vi "HFRR ADV v041.vi"() -> ()   [LabVIEW 2025] (continued)
                n3153 = for {
                  N: 1 -> [_]
                  tunnel: [w3970] -> w3918
                  tunnel: [w3969] -> w3917
                  tunnel: w3932 -> [w3968]
                  tunnel: w3931 -> [w3967]
                  n3154 = call-dynamic "New Report Line.vi"("report in"=w3968, "error in (no error)"=w3967) -> ("report out"=w3970:refnum<class "NI_report.lvclass">, "error out"=w3969:errorcluster)  [unwired: 12 in]
                }
                n3155 = for {
                  N: 2 -> [_]
                  tunnel: [w3962] -> w3924
                  tunnel: [w3961] -> w3923
                  tunnel: w3918 -> [w3960]
                  tunnel: w3917 -> [w3959]
                  n3156 = call-dynamic "New Report Line.vi"("report in"=w3960, "error in (no error)"=w3959) -> ("report out"=w3962:refnum<class "NI_report.lvclass">, "error out"=w3961:errorcluster)  [unwired: 12 in]
                }
                n3157 = for {
                  N: 25 -> [_]
                  tunnel: w3924 -> [w3958]
                  tunnel: w3923 -> [w3956]
                  tunnel: [w3957] -> w3927
                  tunnel: [w3955] -> w3926
                  n3158 = call-dynamic "Set Report Tab Width.vi"("report in"=w3958, "error in (no error)"=w3956) -> ("report out"=w3957:refnum<class "NI_report.lvclass">, "error out"=w3955:errorcluster)  [unwired: 12 in]
                }
                n3159 = control-ref of="Tab Control 9"() -> (w3922:refnum<vi>)
                n3160 = call-dynamic "Append Control Image to Report.vi"("report in"=w3927, "alignment (default)"=HTML_Report_Image_Alignment."ABSMIDDLE", "ctrl reference"=w3922, "error in (no error)"=w3926) -> ("report out"=w3921:refnum<class "NI_report.lvclass">, "error out"=w3920:errorcluster)  [unwired: 8 in, 2 out]
                n3161 = for {
                  N: 3 -> [_]
                  tunnel: [w3954] -> w3905
                  tunnel: [w3953] -> w3904
                  tunnel: w3921 -> [w3952]
                  tunnel: w3920 -> [w3951]
                  n3162 = call-dynamic "New Report Line.vi"("report in"=w3952, "error in (no error)"=w3951) -> ("report out"=w3954:refnum<class "NI_report.lvclass">, "error out"=w3953:errorcluster)  [unwired: 12 in]
                }
                n3163 = for {
                  N: 100 -> [_]
                  tunnel: w3905 -> [w3950]
                  tunnel: w3904 -> [w3948]
                  tunnel: [w3949] -> w3901
                  tunnel: [w3947] -> w3899
                  n3164 = call-dynamic "Set Report Tab Width.vi"("report in"=w3950, "error in (no error)"=w3948) -> ("report out"=w3949:refnum<class "NI_report.lvclass">, "error out"=w3947:errorcluster)  [unwired: 12 in]
                }
                n3165 = String To Path(string="C:\\LAB-IQ\\im\\Temp_resized.jpg") -> (path=w3891:path)
                n3166 = call-poly <vilib>:"Append Image to Report.vi"("report in"=w3901, "path or URL of image"=w3891, "error in (no error)"=w3899) -> ("report out"=w3900:refnum<class "NI_report.lvclass">, "error out"=w3898:errorcluster)  [unwired: 9 in, 2 out]
                n3167 = call-poly <vilib>:"Open HTML Report in Browser.vi"("report in"=w3900, "error in (no error)"=w3898) -> ("report out"=w3935:refnum<class "NI_report.lvclass">, "error out"=w3934:errorcluster)  [unwired: 11 in, 1 out]
                n3168 = call-dynamic "Dispose Report.vi"("report in"=w3935, "error in (no error)"=w3934) -> ()  [unwired: 13 in, 1 out]
              }
              frame #2 {
              }
              frame #3 {
                n3169 = disable-structure shown="Disabled" {
                  frame Disabled {
                    n3170 = local read "String 10"() -> (w3975:string)
                    n3171 = Concatenate Strings("C:\\LAB-IQ-NXT\\Data\\" ("string"), w3975, ".jpg" ("string")) -> (w3973:string)
                    n3172 = String To Path(string=w3973) -> (path=w3972:path)
                    n3173 = Delete(path (use dialog)=w3972) -> ()  [unwired: 4 in, 3 out]
                  }
                  frame Enabled {
                  }
                }
                n3174 = local write "Print 2"(FALSE ("Print")) -> ()
              }
            }
          }
        }
      }
    }
    n3175 = Wait (ms)(milliseconds to wait=u32 50) -> ()  [unwired: 1 out]
    n3176 = Wait (ms)(milliseconds to wait=u32 50) -> ()  [unwired: 1 out]
    n3177 = local read "Quit"() -> (w2317:bool)
  }
  n3178 = VISA Close(VISA resource name=w43, error in (no error)=w42) -> ()  [unwired: 1 out]
  n3179 = while {
    stop <- w4126 stop-if-true
    n3180 = local read "Auto Start Test"() -> (w4124:bool)
    n3181 = local read "RUN"() -> (w4123:bool)
    n3182 = Wait (ms)(milliseconds to wait=u32 1000) -> ()  [unwired: 1 out]
    n3183 = Or(x=w4123, y=w4124) -> (x .or. y?=w4122:bool)
    n3184 = case shown="True" w4122 {
      frame False {
      }
      frame True {
        n3185 = local read "LVDT STROKE Actual"() -> (w4127:dbl)
        n3186 = In Range and Coerce(upper limit=1.2, x=w4127, lower limit=0.6) -> (In Range?=w4130:bool)  [unwired: 1 out]
        n3187 = call-poly <vilib>:"Random Number (Range).vi"("lower bound (0)"=0.998 ("upper bound (100)"), "upper bound (100)"=1.003) -> ("number"=w4128:dbl)  [unwired: 9 in]
        n3188 = case shown="True" w4130 {
          tunnel: [w4135 w4136] -> w4129
          tunnel: w4128 -> [_ w4136]
          tunnel: w4127 -> [w4135 _]
          frame False {
          }
          frame True {
          }
        }
        "LVDT STROKE DISPLAY" <- w4129
      }
    }
    n3189 = local read "Quit"() -> (w4126:bool)
  }
  n3190 = while {
    tunnel: [w4153] -> w51
    shift-right: [w4146] -> _
    shift-left: 0.0 -> [w4149]
    shift-right: [w4145] -> _
    shift-left: 0.0 -> [w4148]
    shift-right: [w4144] -> _
    shift-left: 100.0 ("vc_cmd") -> [w4147]
    stop <- w4153 stop-if-true
    # "PID LOGIC"
    n3191 = local read "run test Calibration"() -> (w4141:bool)
    n3192 = local read "RUN"() -> (w4151:bool)
    n3193 = local read "Auto Start Temp"() -> (w4142:bool)
    n3194 = local read "Auto Start Test"() -> (w4150:bool)
    n3195 = local read "START TEMP"() -> (w4140:bool)
    n3196 = And(x=w4142, y=w4150) -> (x .and. y?=w4143:bool)
    n3197 = Or(x=w4151, y=w4143) -> (x .or. y?=w4152:bool)
    n3198 = And(x=w4152, y=w4140) -> (x .and. y?=w4139:bool)
    n3199 = And(x=w4141, y=w4140) -> (x .and. y?=w4138:bool)
    n3200 = Or(x=w4138, y=w4139) -> (x .or. y?=w4137:bool)
    n3201 = Wait (ms)(milliseconds to wait="milliseconds to wait") -> ()  [unwired: 1 out]
    n3202 = case shown="True" w4137 {
      tunnel: [400.0 ("out_vc_cmd") w4172] -> w4144
      tunnel: [w4156 w4174] -> w4145
      tunnel: [w4156 w4173] -> w4146
      tunnel: w4149 -> [_ w4163]
      tunnel: w4148 -> [_ w4162]
      tunnel: w4147 -> [_ w4161]
      tunnel: w4141 -> [_ w4157]
      frame False {
        w4156 = 0.0 ("error_out")
      }
      frame True {
        n3203 = case shown="True" w4157 {
          tunnel: [w4181 1.0] -> w4159
          frame False {
            n3204 = local read "Set Strk"() -> (w4180:dbl)
            n3205 = Add(x=w4180, y="Add up Stroke") -> (x+y=w4181:dbl)
          }
          frame True {
          }
        }
        n3206 = local read "LVDT STROKE"() -> (w4158:dbl)
        n3207 = formula code="// Zero-Hardcode Explicit Positional-Form PID Engine\n// Inputs: target_stroke, measured_stroke, dt, prev_error, integral_accumulator_in, prev_vc_cmd\n//         kp, ki, kd, max_step_change, max_amplitude, min_amplitude, startup_cmd\n// Outputs: vc_cmd, error_out, out_error, integral_accumulator_out, out_vc_cmd\n\n// 1. Calculate Tracking Error\nfloat current_error = target_stroke - measured_stroke;\nerror_out = current_error;\n\n// 2. Compute Proportional Term\nfloat p_term = kp * current_error;\n\n// 3. Compute Derivative Term\nfloat d_term = 0.0;\nif (dt > 0.0) {\n    d_term = kd * ((current_error - prev_error) / dt);\n}\n\n// 4. Update and Accumulate Integral Term\nfloat current_integral = integral_accumulator_in + (current_error * dt);\nfloat i_term = ki * current_integral;\n\n// 5. Calculate Ideal Target Command (Anchored by startup baseline)\nfloat ideal_command = startup_cmd + p_term + i_term + d_term;\n\n// 6. Apply Loop Rate Limiting FIRST \n// (Forces the command to climb gradually from prev_vc_cmd instead of jumping straight to max)\nfloat raw_adjustment = ideal_command - prev_vc_cmd;\n\nif (raw_adjustment > max_step_change) {\n    raw_adjustment = max_step_change;\n} else if (raw_adjustment < -max_step_change) {\n    raw_adjustment = -max_step_change;\n}\n\nfloat next_vc_cmd = prev_vc_cmd + raw_adjustment;\n\n// 7. Anti-Windup Protection & Final Output Safety Safeguard Clamping\n// (Back-calculating based on what we are ACTUALLY outputting)\nif (next_vc_cmd > max_amplitude) {\n    float excess = next_vc_cmd - max_amplitude;\n    if (ki > 0.0) {\n        current_integral -= excess / ki;\n    }\n    next_vc_cmd = max_amplitude;\n} else if (next_vc_cmd < min_amplitude) {\n    float excess = next_vc_cmd - min_amplitude;\n    if (ki > 0.0) {\n        current_integral -= excess / ki;\n    }\n    next_vc_cmd = min_amplitude;\n}\n\n// 8. Map to Shift Registers for memory persistence\nvc_cmd = next_vc_cmd;\nout_error = current_error;                   \nintegral_accumulator_out = current_integral;  \nout_vc_cmd = next_vc_cmd;"("target_stroke"=w4159, "measured_stroke"=w4158, "dt"="dt", "integral_accumulator_in"=w4162, "prev_error"=w4163, "prev_vc_cmd"=w4161, "kp"="kp", "ki"="ki", "kd"="kd", "max_step_change"="max_step_change", "max_amplitude"="max_amplitude", "min_amplitude"="min_amplitude", "startup_cmd"="startup_cmd") -> ("vc_cmd"=w4178:dbl, "out_error"=w4173:dbl, "integral_accumulator_out"=w4174:dbl, "out_vc_cmd"=w4172:dbl)  [unwired: 1 out]
        "output Vpp" <- w4178
        n3208 = Number To Fractional String(number=w4178, precision (6)=i16 1) -> (F-format string=w4176:string)  [unwired: 2 in]
        n3209 = Concatenate Strings("DAC;" ("string"), w4176) -> (w4160:string)
        n3210 = local write "Due Write"(w4160) -> ()
        "prev_error" <- w4163
        "integral_accumulator_in" <- w4162
        "prev_vc_cmd" <- w4161
      }
    }
    n3211 = local read "Quit"() -> (w4153:bool)
  }
  n3212 = Or(x=w47, y=w46) -> (x .or. y?=w48:bool)
  n3213 = Or(x=w44, y=w48) -> (x .or. y?=w53:bool)
  n3214 = control-ref of="new picture"() -> ()  [unwired: 1 out]
  n3215 = Or(x=w56, y=w53) -> (x .or. y?=w50:bool)
  n3216 = Or(x=w50, y=w51) -> (x .or. y?=w45:bool)
  n3217 = while {
    tunnel: [w4183] -> w55
    i -> [w4190]
    stop <- w4183 stop-if-true
    n3218 = local read "Quit"() -> (w4183:bool)
    n3219 = Equal To 0?(x=w4190) -> (x = 0?=w4188:bool)
    n3220 = call "Elapsed Time3"("Time Target (s)"=45.0, "Auto Reset"=TRUE) -> ("Time has Elapsed"=w4187:bool)  [unwired: 10 in, 7 out]
    n3221 = Wait (ms)(milliseconds to wait=u32 50) -> ()  [unwired: 1 out]
    n3222 = Or(x=w4187, y=w4188) -> (x .or. y?=w4189:bool)
    n3223 = case shown="True" w4189 {
      frame False {
      }
      frame True {
        n3224 = call <vilib>:"System Exec.vi"("run minimized? (F)"=TRUE, "error in (no error)"="error in (no error)", "command line"="powercfg.exe -change -monitor-timeout-ac 0") -> ("error out"=w4201:errorcluster)  [unwired: 5 in, 3 out]
        n3225 = call <vilib>:"System Exec.vi"("run minimized? (F)"=TRUE, "error in (no error)"=w4201, "command line"="powercfg.exe -change -disk-timeout-ac 0") -> ("error out"=w4200:errorcluster)  [unwired: 5 in, 3 out]
        n3226 = call <vilib>:"System Exec.vi"("run minimized? (F)"=TRUE, "error in (no error)"=w4200, "command line"="powercfg.exe -change -standby-timeout-ac 0") -> ("error out"=w4199:errorcluster)  [unwired: 5 in, 3 out]
        n3227 = call <vilib>:"System Exec.vi"("run minimized? (F)"=TRUE, "error in (no error)"=w4199, "command line"="powercfg.exe -change -hibernate-timeout-ac 0") -> ("error out"=w4198:errorcluster)  [unwired: 5 in, 3 out]
        n3228 = call <vilib>:"Simple Error Handler.vi"("error in (no error)"=w4198) -> ("error out"=w4204:errorcluster)  [unwired: 4 in, 4 out]
        n3229 = call <vilib>:"Clear Errors.vi"("error in (no error)"=w4204) -> ("error out"=→"error out":errorcluster)  [unwired: 5 in, 1 out]
      }
    }
  }
  n3230 = Compound Arithmetic op=OR(w58, w45, w55) -> (w57:bool)
  n3231 = flat-sequence {
    tunnel: w57 -> [_]
    tunnel: [w4206] -> w27
    tunnel: w27 -> [_]
    frame #0 {
      n3232 = call "CLOSE CONNECTION.vi"() -> ("error out"=w4206:errorcluster)  [unwired: 11 in]
    }
    frame #1 {
      n3233 = Quit LabVIEW(quit? (T)=TRUE) -> ()
      n3234 = local write "Quit"(FALSE ("EXIT")) -> ()
    }
  }
  n3235 = property on="Heater Button" class="Bool (strict)"("Visible"=TRUE) -> ()  [unwired: 2 in, 2 out]
  n3236 = while {
    tunnel: [w4213] -> _
    i -> [w4213]
    stop <- w4209 stop-if-true
    # "Langauage selection"
    n3237 = Equal?(x="Lan flag", y=22.0) -> ()  [unwired: 1 out]
    n3238 = disable-structure shown="Disabled" {
      frame Disabled {
        n3239 = stacked-sequence {
          frame #0 {
            n3240 = case shown="\"Russian\"" "Language Selection" {
              tunnel: [0 1] -> w4215
              frame "English", Default {
              }
              frame "Russian" {
              }
            }
            n3241 = for {
              N: 130 -> [_]
              tunnel: "Table" -> [w4224]
              tunnel: w4215 -> [w4223]
              i -> [w4222]
              n3242 = Index Array(array=w4224, index (row)=w4222, index (col)=w4223) -> (element=w4221:string)
              n3243 = case shown="1" w4222 {
                tunnel: w4221 -> [w4225 w4226 _ w4227 w4228 w4229 w4230 w4231 w4232 w4233 w4234 w4235 w4236 w4237 w4238 w4239 w4240 w4241 w4242 w4243 w4244 w4245 w4246 w4247 w4248 w4249 w4250 w4251 w4252 _ _ w4253 w4254 w4255 w4256 w4257 w4258 w4267 w4274 w4281 w4288 w4292 w4295 w4298 w4300 w4302 w4303 w4304 w4305 w4306 w4307 w4308 w4309 w4310 w4311 w4312 w4313 w4314 w4315 w4316 w4317 w4318 w4319 w4320 w4321 w4322 w4323 w4324 w4325 w4326 w4327 w4328 w4329 w4330 w4331 w4332 w4333 w4334 w4335 w4336 w4337 w4338 w4339 w4340 w4341 w4342 w4343 w4344 w4345 w4346 w4347 w4348 w4349 w4350 w4351 w4352 w4353 w4354 w4355 w4356 w4357 w4358 w4359 w4360 w4361 _ w4362 w4363 w4364 w4365 w4366 w4367 w4368 w4369 w4370 w4371 w4372 w4373 w4374 _ w4375 w4376 w4377 w4378 w4379 w4380 _]
                frame 0 {
                  n3244 = local write "S"(w4225) -> ()
                }
                frame 1 {
                  n3245 = local write "S 2"(w4226) -> ()
                }
                frame 2 {
                }
                frame 3 {
                  n3246 = local write "S 4"(w4227) -> ()
                }
                frame 4 {
                  n3247 = property on="FILE" class="Str"("Caption.Text"=w4228) -> ()  [unwired: 2 in, 2 out]
                }
                frame 5 {
                  n3248 = property on="Fuel Discription :" class="Str"("Caption.Text"=w4229) -> ()  [unwired: 2 in, 2 out]
                }
                frame 6 {
                  n3249 = property on="Remarks :" class="Str"("Caption.Text"=w4230) -> ()  [unwired: 2 in, 2 out]
                }
                frame 7 {
                  n3250 = property on="Save & Continue" class="Bool (strict)"("Boolean Text.Text"=w4231) -> ()  [unwired: 2 in, 2 out]
                }
                frame 8 {
                }
                frame 9 {
                  n3251 = property on="Set Hz" class="DigNum (strict)"("Caption.Text"=w4233) -> ()  [unwired: 2 in, 2 out]
                }
                frame 10 {
                }
                frame 11 {
                  n3252 = property on="NORMAL LOAD" class="DigNum (strict)"("Caption.Text"=w4235) -> ()  [unwired: 2 in, 2 out]
                }
                frame 12 {
                }
                frame 13 {
                  n3253 = property on="Set Temp" class="DigNum (strict)"("Caption.Text"=w4237) -> ()  [unwired: 2 in, 2 out]
                }
                frame 14 {
                  n3254 = local write "S 15"(w4238) -> ()
                }
                frame 15 {
                  n3255 = property on="Set Rh" class="DigNum (strict)"("Caption.Text"=w4239) -> ()  [unwired: 2 in, 2 out]
                }
                frame 16 {
                }
                frame 17 {
                  n3256 = local write "S 18"(w4241) -> ()
                }
                frame 18 {
                  "String 17" <- w4242
                }
                frame 19 {
                  n3257 = property on="test time" class="DigNum (strict)"("Caption.Text"=w4243) -> ()  [unwired: 2 in, 2 out]
                }
                frame 20 {
                  "String 18" <- w4244
                  "String 22" <- w4244
                }
                frame 21 {
                  n3258 = property on="Elapsed time" class="DigNum (strict)"("Caption.Text"=w4245) -> ()  [unwired: 2 in, 2 out]
                }
                frame 22 {
                  n3259 = property on="Samplingtime 2" class="DigNum (strict)"("Caption.Text"=w4246) -> ()  [unwired: 2 in, 2 out]
                }
                frame 23 {
                  "String 21" <- w4247
                }
                frame 24 {
                  n3260 = property on="Countdown" class="DigNum (strict)"("Caption.Text"=w4248) -> ()  [unwired: 2 in, 2 out]
                }
                frame 25 {
                  n3261 = property on="Countdown 2" class="DigNum (strict)"("Caption.Text"=w4249) -> ()  [unwired: 2 in, 2 out]
                }
                frame 26 {
                  n3262 = property on="Engage" class="Bool (strict)"("Boolean Text.Text"=w4250) -> ()  [unwired: 2 in, 2 out]
                }
                frame 27 {
                  n3263 = property on="Boolean  4" class="Bool (strict)"("Boolean Text.Text"=w4251) -> ()  [unwired: 2 in, 2 out]
                }
                frame 28 {
                  n3264 = property on="Test \nStatus" class="Bool (strict)"("Boolean Text.Text"=w4252) -> ()  [unwired: 2 in, 2 out]
                }
                frame 29 {
                }
                frame 30 {
                }
                frame 31 {
                }
                frame 32 {
                  n3265 = property on="RSTCOF" class="Bool"("Boolean Text.Text"=w4254) -> ()  [unwired: 2 in, 2 out]
                  n3266 = property on="RST FF" class="Bool"("Boolean Text.Text"=w4254) -> ()  [unwired: 2 in, 2 out]
                  n3267 = property on="RST TEMP" class="Bool"("Boolean Text.Text"=w4254) -> ()  [unwired: 2 in, 2 out]
                  n3268 = property on="RSTV1 3" class="Bool"("Boolean Text.Text"=w4254) -> ()  [unwired: 2 in, 2 out]
                  n3269 = property on="rstv2" class="Bool"("Boolean Text.Text"=w4254) -> ()  [unwired: 2 in, 2 out]
                  n3270 = property on="RSTV1 2" class="Bool"("Boolean Text.Text"=w4254) -> ()  [unwired: 2 in, 2 out]
                  n3271 = property on="RST CP" class="Bool"("Boolean Text.Text"=w4254) -> ()  [unwired: 2 in, 2 out]
                }
                frame 33 {
                  "S 61" <- w4255
                }
                frame 34 {
                  "String 23" <- w4256
                }
                frame 35 {
                  n3272 = property on="Rh Before" class="DigNum (strict)"("Caption.Text"=w4257) -> ()  [unwired: 2 in, 2 out]
                }
                frame 36 {
                  n3273 = Match Pattern(string=w4258, regular expression=",") -> (before substring=→"bs":string, after substring=→"as":string)  [unwired: 1 in, 2 out]
                  n3274 = property on="Rh After" class="DigNum (strict)"("Caption.Text"=w4258) -> ()  [unwired: 2 in, 2 out]
                }
                frame 37 {
                  n3275 = Match Pattern(string=w4267, regular expression=",") -> (before substring=w4266:string, after substring=w4265:string)  [unwired: 1 in, 2 out]
                  "bs" <- w4266
                  "as" <- w4265
                  n3276 = Concatenate Strings(w4266, w4265) -> (w4262:string)
                  n3277 = property on="Humidity before test 2" class="DigNum (strict)"("Caption.Text"=w4262) -> ()  [unwired: 2 in, 2 out]
                  n3278 = Concatenate Strings(w4262, "=" ("string")) -> (w4263:string)
                  n3279 = local write "S 38"(w4263) -> ()
                }
                frame 38 {
                  n3280 = Match Pattern(string=w4274, regular expression=",") -> (before substring=w4273:string, after substring=w4272:string)  [unwired: 1 in, 2 out]
                  "bs" <- w4273
                  "as" <- w4272
                  n3281 = Concatenate Strings(w4273, w4272) -> (w4269:string)
                  n3282 = property on="Humidity after test 2" class="DigNum (strict)"("Caption.Text"=w4269) -> ()  [unwired: 2 in, 2 out]
                  n3283 = Concatenate Strings(w4269, "=" ("string")) -> (w4271:string)
                  n3284 = local write "S 39"(w4271) -> ()
                }
                frame 39 {
                  n3285 = Match Pattern(string=w4281, regular expression=",") -> (before substring=w4280:string, after substring=w4279:string)  [unwired: 1 in, 2 out]
                  "bs" <- w4280
                  "as" <- w4279
                  n3286 = Concatenate Strings(w4280, w4279) -> (w4276:string)
                  n3287 = property on="Temperature before test 2" class="DigNum (strict)"("Caption.Text"=w4276) -> ()  [unwired: 2 in, 2 out]
                  n3288 = Concatenate Strings(w4276, "=" ("string")) -> (→"String 34":string)
                }
                frame 40 {
                  n3289 = Match Pattern(string=w4288, regular expression=",") -> (before substring=w4287:string, after substring=w4286:string)  [unwired: 1 in, 2 out]
                  "bs" <- w4287
                  "as" <- w4286
                  n3290 = Concatenate Strings(w4287, w4286) -> (w4283:string)
                  n3291 = property on="Temperature after test 2" class="DigNum (strict)"("Caption.Text"=w4283) -> ()  [unwired: 2 in, 2 out]
                  n3292 = Concatenate Strings(w4283, "=" ("string")) -> (→"String 35":string)
                  n3293 = property on="Temperature after test" class="DigNum (strict)"("Caption.Text"=w4283) -> ()  [unwired: 2 in, 2 out]
                }
                frame 41 {
                  n3294 = property on="AVP 2" class="DigNum (strict)"("Caption.Text"=w4292) -> ()  [unwired: 2 in, 2 out]
                  n3295 = Concatenate Strings(w4292, "=" ("string")) -> (→"String 36":string)
                }
                frame 42 {
                  n3296 = property on="MWSD 2" class="DigNum (strict)"("Caption.Text"=w4295) -> ()  [unwired: 2 in, 2 out]
                  n3297 = Concatenate Strings(w4295, "=" ("string")) -> (→"String 37":string)
                }
                frame 43 {
                  n3298 = property on="HCF 2" class="DigNum (strict)"("Caption.Text"=w4298) -> ()  [unwired: 2 in, 2 out]
                  n3299 = Concatenate Strings(w4298, "=" ("string")) -> (→"String 38":string)
                }
                frame 44 {
                  n3300 = Concatenate Strings(w4300, "=" ("string")) -> (→"String 39":string)
                  n3301 = property on="WS1.4 2" class="DigNum (strict)"("Caption.Text"=w4300) -> ()  [unwired: 2 in, 2 out]
                }
                frame 45 {
                }
                frame 46 {
                  n3302 = local write "S 47"(w4303) -> ()
                }
                frame 47 {
                  n3303 = local write "S 48"(w4304) -> ()
                }
                frame 48 {
                  n3304 = local write "S 49"(w4305) -> ()
                }
                frame 49 {
                  n3305 = local write "S 50"(w4306) -> ()
                }
                frame 50 {
                  n3306 = local write "S 51"(w4307) -> ()
                }
                frame 51 {
                  n3307 = local write "S 52"(w4308) -> ()
                }
                frame 52 {
                  n3308 = local write "S 53"(w4309) -> ()
                }
                frame 53 {
                  n3309 = local write "S 54"(w4310) -> ()
                }
                frame 54 {
                  n3310 = local write "S 55"(w4311) -> ()
                }
                frame 55 {
                  n3311 = local write "S 56"(w4312) -> ()
                }
                frame 56 {
                  n3312 = local write "S 57"(w4313) -> ()
                }
                frame 57 {
                  n3313 = local write "S 58"(w4314) -> ()
                }
                frame 58 {
                  n3314 = local write "S 59"(w4315) -> ()
                }
                frame 59 {
                  n3315 = local write "S 60"(w4316) -> ()
                }
                frame 60 {
                  n3316 = local write "S 62"(w4317) -> ()
                }
                frame 61 {
                  n3317 = local write "S 63"(w4318) -> ()
                }
                frame 62 {
                  n3318 = local write "S 64"(w4319) -> ()
                }
                frame 63 {
                  n3319 = local write "S 65"(w4320) -> ()
                }
                frame 64 {
                  n3320 = local write "S 66"(w4321) -> ()
                }
                frame 65 {
                  n3321 = local write "S 67"(w4322) -> ()
                }
                frame 66 {
                  n3322 = local write "S 68"(w4323) -> ()
                }
                frame 67 {
                  n3323 = local write "S 69"(w4324) -> ()
                }
                frame 68 {
                  n3324 = local write "S 70"(w4325) -> ()
                }
                frame 69 {
                  n3325 = local write "S 71"(w4326) -> ()
                }
                frame 70 {
                  n3326 = local write "S 72"(w4327) -> ()
                }
                frame 71 {
                  n3327 = local write "S 73"(w4328) -> ()
                }
                frame 72 {
                  n3328 = local write "S 74"(w4329) -> ()
                }
                frame 73 {
                  n3329 = local write "S 75"(w4330) -> ()
                }
                frame 74 {
                  n3330 = local write "S 76"(w4331) -> ()
                }
                frame 75 {
                  n3331 = local write "S 77"(w4332) -> ()
                }
                frame 76 {
                  n3332 = local write "S 78"(w4333) -> ()
                }
                frame 77 {
                  n3333 = local write "S 79"(w4334) -> ()
                }
                frame 79 {
                  n3334 = property on="Sample Temperature ( °C )" class="XYGraph (strict)"("Y Scale.Name Label.Text"=w4335) -> ()  [unwired: 2 in, 2 out]
                }
                frame 80 {
                  n3335 = local write "S 81"(w4336) -> ()
                  n3336 = property on="Humidity ( %RH )" class="XYGraph (strict)"("Y Scale.Name Label.Text"=w4336) -> ()  [unwired: 2 in, 2 out]
                }
                frame 78 {
                  n3337 = property on="Air Temperature  ( °C )" class="XYGraph (strict)"("X Scale.Name Label.Text"=w4337) -> ()  [unwired: 2 in, 2 out]
                  n3338 = property on="Humidity ( %RH )" class="XYGraph (strict)"("X Scale.Name Label.Text"=w4337) -> ()  [unwired: 2 in, 2 out]
                  n3339 = property on="Sample Temperature ( °C )" class="XYGraph (strict)"("X Scale.Name Label.Text"=w4337) -> ()  [unwired: 2 in, 2 out]
                  n3340 = property on="Coefficient Of Friction" class="XYGraph (strict)"("X Scale.Name Label.Text"=w4337) -> ()  [unwired: 2 in, 2 out]
                }
                frame 81 {
                  n3341 = property on="Air Temperature  ( °C )" class="XYGraph (strict)"("Y Scale.Name Label.Text"=w4338) -> ()  [unwired: 2 in, 2 out]
                }
                frame 82 {
                  n3342 = local write "S 84"(w4339) -> ()
                }
                frame 83 {
                  n3343 = local write "S 85"(w4340) -> ()
                }
                frame 84 {
                  n3344 = local write "S 86"(w4341) -> ()
                }
                frame 85 {
                  n3345 = local write "S 87"(w4342) -> ()
                }
                frame 86 {
                  n3346 = local write "S 88"(w4343) -> ()
                }
                frame 87 {
                }
                frame 88 {
                  n3347 = local write "S 90"(w4345) -> ()
                }
                frame 89 {
                  n3348 = local write "S 91"(w4346) -> ()
                }
                frame 90 {
                  n3349 = local write "S 92"(w4347) -> ()
                }
                frame 91 {
                  n3350 = local write "S 93"(w4348) -> ()
                }
                frame 92 {
                  n3351 = local write "S 94"(w4349) -> ()
                }
                frame 93 {
                  n3352 = local write "S 95"(w4350) -> ()
                }
                frame 94 {
                  n3353 = local write "S 96"(w4351) -> ()
                }
                frame 95 {
                  n3354 = local write "S 97"(w4352) -> ()
                }
                frame 96 {
                  n3355 = local write "S 98"(w4353) -> ()
                }
                frame 97 {
                  n3356 = local write "S 99"(w4354) -> ()
                }
                frame 98 {
                  n3357 = local write "S 100"(w4355) -> ()
                }
                frame 99 {
                  n3358 = local write "S 101"(w4356) -> ()
                }
                frame 100 {
                  n3359 = local write "S 102"(w4357) -> ()
                }
                frame 101 {
                  n3360 = local write "S 103"(w4358) -> ()
                }
                frame 102 {
                  n3361 = local write "S 104"(w4359) -> ()
                }
                frame 103 {
                  n3362 = local write "S 105"(w4360) -> ()
                }
                frame 104 {
                  n3363 = local write "S 106"(w4361) -> ()
                }
                frame 105 {
                }
                frame 106 {
                  n3364 = property on="OK Button 17" class="Bool (strict)"("Boolean Text.Text"=w4362) -> ()  [unwired: 2 in, 2 out]
                }
                frame 107 {
                  n3365 = property on="OK Button 16" class="Bool (strict)"("Boolean Text.Text"=w4363) -> ()  [unwired: 2 in, 2 out]
                }
                frame 108 {
                  n3366 = property on="TITTLE" class="Str"("Caption.Text"=w4364) -> ()  [unwired: 2 in, 2 out]
                }
                frame 109 {
                  "String 30" <- w4365
                }
                frame 110 {
                  n3367 = property on="Test Date" class="Str"("Caption.Text"=w4366) -> ()  [unwired: 2 in, 2 out]
                  "String 31" <- w4366
                }
                frame 111 {
                  n3368 = property on="Sample ID" class="Str"("Caption.Text"=w4367) -> ()  [unwired: 2 in, 2 out]
                  "String 32" <- w4367
                }
                frame 112 {
                  n3369 = property on="Tested by" class="Str"("Caption.Text"=w4368) -> ()  [unwired: 2 in, 2 out]
                  "String 33" <- w4368
                }
                frame 113 {
                  n3370 = property on="System Configured Printers 2" class="Arr (strict)"("Caption.Text"=w4369) -> ()  [unwired: 2 in, 2 out]
                }
                frame 114 {
                  n3371 = property on="Selected Printer" class="Str"("Caption.Text"=w4370) -> ()  [unwired: 2 in, 2 out]
                }
                frame 115 {
                  n3372 = property on="Select Printer 3" class="DigNum (strict)"("Caption.Text"=w4371) -> ()  [unwired: 2 in, 2 out]
                }
                frame 116 {
                  n3373 = property on="Print" class="Bool (strict)"("Boolean Text.Text"=w4372) -> ()  [unwired: 2 in, 2 out]
                }
                frame 117 {
                  "String 41" <- w4373
                }
                frame 118 {
                  n3374 = property on="tested by" class="Str"("Caption.Text"=w4374) -> ()  [unwired: 2 in, 2 out]
                }
                frame 119 {
                }
                frame 120 {
                  n3375 = property on="Export" class="Bool (strict)"("Boolean Text.Text"=w4375) -> ()  [unwired: 2 in, 2 out]
                }
                frame 121 {
                }
                frame 122 {
                }
                frame 123 {
                  n3376 = property on="Select File Type" class="Enum (strict)"("Caption.Text"=w4378) -> ()  [unwired: 2 in, 2 out]
                }
                frame 124 {
                  n3377 = property on="s.NO" class="Str"("Caption.Text"=w4379) -> ()  [unwired: 2 in, 2 out]
                  "String 45" <- w4379
                }
                frame 125 {
                  n3378 = property on="trip1 8" class="Bool (strict)"("Boolean Text.Text"=w4380) -> ()  [unwired: 2 in, 2 out]
                }
                frame 126, Default {
                }
              }
            }
          }
          frame #1 {
            w4388 = TRUE ("Visible")
            n3379 = local read "S 91"() -> (w4405:string)
            n3380 = local read "S 90"() -> (w4404:string)
            n3381 = local read "S 88"() -> (w4403:string)
            n3382 = property on="File Path" class="Path"("Caption.Text"=w4404) -> ()  [unwired: 2 in, 2 out]
            n3383 = local read "S 71"() -> (w4398:string)
            n3384 = local read "S 86"() -> (w4400:string)
            n3385 = local read "S 85"() -> (w4401:string)
            n3386 = local read "S 87"() -> (w4399:string)
            n3387 = local read "S 84"() -> (w4402:string)
            n3388 = local read "S 103"() -> (w4387:string)
            n3389 = local read "S 104"() -> (w4386:string)
            n3390 = property on="Password" class="Str"("Caption.Text"=w4401) -> ()  [unwired: 2 in, 2 out]
            n3391 = property on="EDIT" class="Bool (strict)"("Boolean Text.Text"=w4398) -> ()  [unwired: 2 in, 2 out]
            n3392 = property on="SAVE" class="Bool (strict)"("Boolean Text.Text"=w4402) -> ()  [unwired: 2 in, 2 out]
            n3393 = Build Array(w4387, w4386) -> (w4385:string[])
            n3394 = property on="Heater Button" class="Bool (strict)"("Strings [4]"=w4385) -> ()  [unwired: 2 in, 2 out]
            n3395 = local read "S 92"() -> (w4397:string)
            n3396 = local read "S 93"() -> (w4396:string)
            n3397 = local read "S 105"() -> (w4383:string)
            n3398 = local read "S 106"() -> (w4382:string)
            n3399 = Build Array(w4397, w4396) -> ()  [unwired: 1 out]
            n3400 = Build Array(w4383, w4382) -> (w4384:string[])
            n3401 = local read "S 95"() -> (w4394:string)
            n3402 = local read "S 94"() -> (w4395:string)
            n3403 = local read "bs"() -> (w4410:string)
            n3404 = local read "as"() -> (w4411:string)
            n3405 = property on="Humidity" class="Bool (strict)"("Strings [4]"=w4384) -> ()  [unwired: 2 in, 2 out]
            n3406 = Concatenate Strings(w4410, "\r", w4411) -> ()  [unwired: 1 out]
            n3407 = property on="Rh After" class="DigNum (strict)"("Caption.Size to Text?"=TRUE ("Caption.Size to Text")) -> ()  [unwired: 2 in, 2 out]
            n3408 = local read "S 48"() -> (w4434:string)
            n3409 = local read "S 50"() -> (w4432:string)
            n3410 = local read "S 51"() -> (w4431:string)
            n3411 = local read "S 49"() -> (w4433:string)
            n3412 = local read "S 52"() -> (w4430:string)
            n3413 = local read "as"() -> (w4415:string)
            n3414 = local read "bs"() -> (w4416:string)
            n3415 = local read "S 56"() -> (w4429:string)
            n3416 = local read "S 57"() -> (w4428:string)
            n3417 = local read "S 58"() -> (w4427:string)
            n3418 = local read "S 59"() -> (w4426:string)
            n3419 = property on="OPEN" class="Bool (strict)"("Boolean Text.Text"=w4430) -> ()  [unwired: 2 in, 2 out]
            n3420 = property on="OPEN 1" class="Bool (strict)"("Boolean Text.Text"=w4434) -> ()  [unwired: 2 in, 2 out]
            n3421 = property on="OPEN 2" class="Bool (strict)"("Boolean Text.Text"=w4433) -> ()  [unwired: 2 in, 2 out]
            n3422 = property on="OPEN 3" class="Bool (strict)"("Boolean Text.Text"=w4432) -> ()  [unwired: 2 in, 2 out]
            n3423 = property on="OPEN 4" class="Bool (strict)"("Boolean Text.Text"=w4431) -> ()  [unwired: 2 in, 2 out]
            n3424 = Concatenate Strings(w4416, "\r", w4415) -> ()  [unwired: 1 out]
            n3425 = local read "S 102"() -> (w4389:string)
            n3426 = property on="КОФ1" class="DigNum (strict)"("Caption.Text"=w4429) -> ()  [unwired: 2 in, 2 out]
            n3427 = local read "S 98"() -> (w4393:string)
            n3428 = local read "S 99"() -> (w4392:string)
            n3429 = local read "S 100"() -> (w4391:string)
            n3430 = local read "S 101"() -> (w4390:string)
            n3431 = property on="КОФ2" class="DigNum (strict)"("Caption.Text"=w4428) -> ()  [unwired: 2 in, 2 out]
            n3432 = property on="КОФ3" class="DigNum (strict)"("Caption.Text"=w4427) -> ()  [unwired: 2 in, 2 out]
            n3433 = property on="КОФ4" class="DigNum (strict)"("Caption.Text"=w4426) -> ()  [unwired: 2 in, 2 out]
            n3434 = local read "bs"() -> (w4414:string)
            n3435 = local read "as"() -> (w4413:string)
            n3436 = local read "S 60"() -> (w4425:string)
            n3437 = local read "S 54"() -> (w4435:string)
            n3438 = Concatenate Strings(w4414, "\r", w4413) -> ()  [unwired: 1 out]
            n3439 = Concatenate Strings(w4435, w4425) -> ()  [unwired: 1 out]
            n3440 = local read "S 77"() -> (→"String 43":string)
            n3441 = local read "S 76"() -> (w4408:string)
            n3442 = local read "S 78"() -> (w4407:string)
            n3443 = local read "S 71"() -> (w4419:string)
            n3444 = local read "S 66"() -> (w4424:string)
            n3445 = local read "S 67"() -> (w4423:string)
            n3446 = local read "S 68"() -> (w4422:string)
            n3447 = local read "S 69"() -> (w4421:string)
            n3448 = local read "S 70"() -> (w4420:string)
            n3449 = property on="AIR TEMP" class="DigNum (strict)"("Caption.Text"=w4407) -> ()  [unwired: 2 in, 2 out]
            n3450 = property on="Set Strk" class="DigNum (strict)"("Caption.Text"=w4408) -> ()  [unwired: 2 in, 2 out]
            n3451 = property on="SPEED OUT:" class="DigNum (strict)"("Caption.Text"=w4422) -> ()  [unwired: 2 in, 2 out]
            n3452 = property on="EDIT" class="Bool (strict)"("Boolean Text.Text"=w4419) -> ()  [unwired: 2 in, 2 out]
            n3453 = local read "S 79"() -> (w4406:string)
          }
          frame #2 {
          }
        }
        n3454 = local write "Lan flag"(10.0 ("Lan flag")) -> ()
      }
      frame Enabled {
      }
    }
    n3455 = Wait (ms)(milliseconds to wait=u32 2000) -> ()  [unwired: 1 out]
    n3456 = local read "Quit"() -> (w4209:bool)
  }
  n3457 = while {
    shift-right: [w4441] -> _
    shift-left: _ -> [w4442]
    shift-right: [w4439] -> _
    shift-left: T18 {"Read Heave and Surge"="", "Bytes at Heave Port"=0.0, "Heave and Surge COM Port:"="COM9", "Com Port 2"="COM7", "Residual Due"="", "Heave COM Status 2"=TRUE, "Heave COM Status"=TRUE, "Port 2"=TRUE, "Sway PPR"=6400.0, "Surge PPR"=6400.0, "Heave PPR"=6400.0, "Sway Pitch"=2.0, "Surge Pitch"=3.0, "Heave Pitch"=4.0, "Sway Pulses/mm"=320.0, "Surge Pulses/mm"=1600.0, "Heave Pulses/mm"=1600.0, "inner loop"=0.0, "Read Heave and Surge 2"="", "String 36"="", "Write S"=FALSE, "WriteCC1"=[""], "Heave COM Loop"=0, "LastCom"="", "EXIT"=FALSE, "Error Heave"={"status"=TRUE, "code"=-1073807343, "source"=""}} -> [w4438]
    shift-right: [w4436] -> _
    shift-left: enum16{"init", "MAIN", "Panel Close"}."init" -> [w4437]
    stop <- w4440 stop-if-true
    # "HUMIDITY LOOP LOGIC"
    n3458 = case shown="\"MAIN\"" w4437 {
      tunnel: w4442 -> [w4456 w4480 w4544 w4546]
      tunnel: [w4451 w4467 w4544 w4546] -> w4441
      tunnel: [_ _ TRUE _] -> w4440
      tunnel: [w4448 w4465 w4542 w4545] -> w4439
      tunnel: w4438 -> [w4453 w4479 w4542 w4545]
      tunnel: [enum16{"init", "MAIN", "Panel Close"}."MAIN" w4474 _ _] -> w4436
      frame "init" {
        n3459 = local read "C3 :"() -> (w4443:refnum<visa-resource-name>)
        n3460 = Bundle By Name(cluster=w4453, "Heave and Surge COM Port:"=w4443) -> (w4452:T18)
        n3461 = call "Instrument fgv uno.vi"("Enum"=T32."INIT", "error in (no error) 2"=w4456, "INPUT"=w4452) -> ("error"=w4454:errorcluster, "output"=w4450:T18)  [unwired: 6 in, 1 out]
        n3462 = case shown="Error" w4454 {
          selector: w4454 -> [w4458 _]
          tunnel: [w4458 w4462] -> w4451
          tunnel: w4450 -> [w4457 w4460]
          tunnel: [w4457 w4459] -> w4449
          frame No Error {
          }
          frame Error {
            n3463 = call "Instrument fgv uno.vi"("Enum"=T32."ERROR INIT", "INPUT"=w4460) -> ("error"=w4463:errorcluster, "output"=w4459:T18)  [unwired: 7 in, 1 out]
            n3464 = call <vilib>:"Clear Errors.vi"("error in (no error)"=w4463) -> ("error out"=w4462:errorcluster)  [unwired: 5 in, 1 out]
          }
        }
        n3465 = local read "LastCom Humidity"() -> (w4446:string)
        n3466 = Unbundle By Name(w4449) -> ("Heave COM Status 2"=→"COM Status":bool, "Error Heave"=→"Error":errorcluster)  [unwired: 1 out]
        n3467 = Bundle By Name(cluster=w4449, "LastCom"=w4446) -> (w4448:T18)
      }
      frame "MAIN" {
        n3468 = Unbundle By Name(w4479) -> ("Com Port 2"=w4469:refnum<visa-resource-name>)
        n3469 = local read "C3 :"() -> (w4470:refnum<visa-resource-name>)
        n3470 = local write "COM Port Humidity :"(w4469) -> ()
        n3471 = Bundle By Name(cluster=w4479, "Heave and Surge COM Port:"=w4470) -> (w4478:T18)
        n3472 = Equal?(x=w4469, y=w4470) -> (x = y?=w4483:bool)
        n3473 = case shown="True" w4483 {
          tunnel: [w4498 w4515] -> w4468
          tunnel: w4480 -> [w4499 w4521]
          tunnel: w4478 -> [w4497 w4519]
          tunnel: [w4496 w4514] -> w4466
          frame False {
            n3474 = call <vilib>:"Clear Errors.vi"("error in (no error)"=w4499) -> ("error out"=w4495:errorcluster)  [unwired: 5 in, 1 out]
            n3475 = call "Instrument fgv uno.vi"("Enum"=T32."ERROR INIT", "error in (no error) 2"=w4495, "INPUT"=w4497) -> ("error"=w4501:errorcluster, "output"=w4496:T18)  [unwired: 6 in, 1 out]
            n3476 = call <vilib>:"Clear Errors.vi"("error in (no error)"=w4501) -> ("error out"=w4498:errorcluster)  [unwired: 5 in, 1 out]
          }
          frame True {
            n3477 = call "Instrument fgv uno.vi"("Enum"=T32."READ", "error in (no error) 2"=w4521, "INPUT"=w4519) -> ("error"=w4520:errorcluster, "output"=w4513:T18)  [unwired: 6 in, 1 out]
            n3478 = Bundle By Name(cluster=w4513, "String 36"="WRITE HUMIDITY") -> (w4512:T18)
            n3479 = case shown="True" "Write Humidity" {
              selector: "Write Humidity" -> [_ w4541]
              tunnel: w4520 -> [w4534 w4540]
              tunnel: [w4534 w4539] -> w4510
              tunnel: w4512 -> [w4533 w4537]
              tunnel: [w4533 w4536] -> w4509
              frame False {
              }
              frame True {
                n3480 = Not(x=w4541) -> (.not. x?=w4535:bool)
                n3481 = local write "Write Humidity"(w4535) -> ()
                n3482 = call "Instrument fgv uno.vi"("Enum"=T32."MANUAL WRITE", "error in (no error) 2"=w4540, "INPUT"=w4537) -> ("error"=w4539:errorcluster, "output"=w4536:T18)  [unwired: 6 in, 1 out]
              }
            }
            n3483 = Array Size(array="WriteHumidity") -> (size(s)=w4507:i32)
            n3484 = Greater Than 0?(x=w4507) -> (x > 0?=w4506:bool)
            n3485 = call "Instrument fgv uno.vi"("Enum"=T32."WRITE", "error in (no error) 2"=w4510, "WriteCC1"="WriteHumidity", "INPUT"=w4509) -> ("error"=w4517:errorcluster, "WriteCC1 2"=w4508:string[], "output"=w4516:T18)  [unwired: 5 in]
            n3486 = case shown="True" w4506 {
              tunnel: w4508 -> [_ w4523]
              frame False {
              }
              frame True {
                n3487 = local write "WriteHumidity"(w4523) -> ()
              }
            }
            n3488 = case shown="No Error" w4517 {
              selector: w4517 -> [w4524 w4527]
              tunnel: w4516 -> [w4525 w4532]
              tunnel: [w4525 w4531] -> w4514
              tunnel: [w4524 w4529] -> w4515
              frame No Error {
              }
              frame Error {
                n3489 = call <vilib>:"Clear Errors.vi"("error in (no error)"=w4527) -> ("error out"=w4526:errorcluster)  [unwired: 5 in, 1 out]
                n3490 = call "Instrument fgv uno.vi"("Enum"=T32."ERROR INIT", "error in (no error) 2"=w4526, "INPUT"=w4532) -> ("error"=w4530:errorcluster, "output"=w4531:T18)  [unwired: 6 in, 1 out]
                n3491 = call <vilib>:"Clear Errors.vi"("error in (no error)"=w4530) -> ("error out"=w4529:errorcluster)  [unwired: 5 in, 1 out]
              }
            }
            n3492 = Unbundle By Name(w4514) -> ("LastCom"=→"LastCom Humidity":string, "Read Heave and Surge"=→"Read HUMIDITY":string)
          }
        }
        n3493 = Unbundle By Name(w4466) -> ("Heave COM Status 2"=w4482:bool, "Error Heave"=w4471:errorcluster, "Bytes at Heave Port"=→"Bytes at Humidity Port  2":dbl)  [unwired: 1 out]
        n3494 = Unbundle By Name(w4471) -> ("status"=→"Humidity Port":bool)
        n3495 = Not(x=w4482) -> (.not. x?=w4472:bool)
        n3496 = local write "Error"(w4471) -> ()
        n3497 = local read "Quit"() -> (w4475:bool)
        n3498 = local write "COM Status"(w4472) -> ()
        n3499 = Select(t=enum16{"init", "MAIN", "Panel Close"}."Panel Close", s=w4475, f=enum16{"init", "MAIN", "Panel Close"}."MAIN") -> (s? t:f=w4474:enum16{"init", "MAIN", "Panel Close"})
        n3500 = local read "Humidity 2"() -> (w4464:bool)
        n3501 = case shown="True" w4464 {
          selector: w4464 -> [_ w4486]
          tunnel: w4468 -> [w4484 w4491]
          tunnel: [w4484 w4490] -> w4467
          tunnel: w4466 -> [w4485 w4489]
          tunnel: [w4485 w4488] -> w4465
          frame False {
          }
          frame True {
            n3502 = Not(x=w4486) -> (.not. x?=→"Humidity 2":bool)
            n3503 = call <vilib>:"Clear Errors.vi"("error in (no error)"=w4491) -> ("error out"=w4494:errorcluster)  [unwired: 5 in, 1 out]
            n3504 = call "Instrument fgv uno.vi"("Enum"=T32."ERROR INIT", "error in (no error) 2"=w4494, "INPUT"=w4489) -> ("error"=w4492:errorcluster, "output"=w4488:T18)  [unwired: 6 in, 1 out]
            n3505 = call <vilib>:"Clear Errors.vi"("error in (no error)"=w4492) -> ("error out"=w4490:errorcluster)  [unwired: 5 in, 1 out]
          }
        }
      }
      frame "Panel Close" {
      }
      frame Default {
      }
    }
  }
  n3506 = while {
    stop <- w4548 stop-if-true
    n3507 = call <vilib>:"High Resolution Polling Wait.vi"("seconds to wait"=0.05) -> ()  [unwired: 10 in, 1 out]
    n3508 = disable-structure shown="Enabled" {
      frame Disabled {
        n3509 = local read "Read HUMIDITY"() -> (w4549:string)
        n3510 = Spreadsheet String To Array(delimiter (Tab)=",", format string="", spreadsheet string=w4549, array type (2D Dbl)=string[] []) -> (array=w4568:string[])
        n3511 = for {
          tunnel: w4568 -> [w4577] mode=indexing
          tunnel: string[] ["STATE;", "SET;", "RH;", "T;", "AMB_RH;", "AMB_T;", "PUMP;", "FAN_IN;", "FAN_OUT;", "DEHUM;", "CURRENT;", "STALL;"] -> [w4576] mode=indexing
          tunnel: [w4575] -> w4567 mode=indexing
          n3512 = Match Pattern(string=w4577, regular expression=w4576) -> (after substring=w4575:string)  [unwired: 1 in, 3 out]
        }
        n3513 = Index Array(array=w4567) -> (element #1=w4566:string, element #2=w4565:string, element #3=w4557:string, element #4=w4556:string, element #5=w4555:string, element #6=w4564:string, element #7=w4563:string, element #8=w4562:string, element #9=w4561:string, element #10=w4560:string, element #11=w4559:string, element #12=w4558:string)  [unwired: 12 in]
        n3514 = Fract/Exp String To Number(string=w4557) -> (number=w4550:dbl)  [unwired: 3 in, 1 out]
        n3515 = Fract/Exp String To Number(string=w4555) -> (number=w4554:dbl)  [unwired: 3 in, 1 out]
        n3516 = local write "Ambient Humidity :"(w4554) -> ()
        n3517 = Equal?(x=w4550, y=0.0) -> (x = y?=w4552:bool)
        n3518 = case shown="True" w4552 {
          tunnel: [w4573 w4574] -> w4551
          tunnel: w4550 -> [w4573 _]
          frame False {
            (unwired) 0.0
            "Humidity temp" <- w4573
          }
          frame True {
            n3519 = local read "Humidity temp"() -> (w4574:dbl)
          }
        }
        "RH Numeric:" <- w4551
      }
      frame Enabled {
        n3520 = local read "Read HUMIDITY"() -> (w4597:string)
        n3521 = Spreadsheet String To Array(delimiter (Tab)=",", format string="", spreadsheet string=w4597, array type (2D Dbl)=dbl[] []) -> (array=w4593:dbl[])
        n3522 = Index Array(array=w4593) -> (element #1=→"STATE :":dbl, element #2=→"SET :":dbl, element #3=w4578:dbl, element #4=→"T :":dbl, element #5=→"AMB_RH :":dbl, element #6=→"AMB_T :":dbl, element #7=→"PUMP :":dbl, element #8=→"FAN_IN :":dbl, element #9=→"FAN_OUT :":dbl, element #10=→"DEHUM :":dbl, element #11=→"CURRENT :":dbl, element #12=→"STALL":dbl)  [unwired: 12 in]
        "RH :" <- w4578
        n3523 = Equal?(x=w4578, y=0.0) -> (x = y?=w4581:bool)
        n3524 = case shown="False" w4581 {
          tunnel: [w4598 w4599] -> w4582
          tunnel: w4578 -> [w4598 _]
          frame False {
            "Humidity temp 2" <- w4598
          }
          frame True {
            n3525 = local read "Humidity temp 2"() -> (w4599:dbl)
          }
        }
        n3526 = local write "RH Numeric:"(w4582) -> ()
      }
    }
    n3527 = local read "Quit"() -> (w4548:bool)
  }
  n3528 = while {
    shift-right: [w4605] -> _
    shift-left: _ -> [w4606]
    shift-right: [w4603] -> _
    shift-left: T20 {"Read Uno"="", "Bytes at Heave Port"=0.0, "UNO COM Port:"="COM9", "UNO COM Port: 2"="COM7", "Residual Due"="", "UNO COM Status 2"=TRUE, "UNO COM Status"=TRUE, "Port 2"=TRUE, "Sway PPR"=6400.0, "Surge PPR"=6400.0, "Heave PPR"=6400.0, "Sway Pitch"=2.0, "Surge Pitch"=3.0, "Heave Pitch"=4.0, "Sway Pulses/mm"=320.0, "Surge Pulses/mm"=1600.0, "Heave Pulses/mm"=1600.0, "inner loop"=0.0, "Read Heave and Surge 2"="", "String 36"="", "Write S"=FALSE, "WriteCC1"=[""], "Heave COM Loop"=0, "LastCom"="", "EXIT"=FALSE, "Error Heave"={"status"=TRUE, "code"=-1073807343, "source"=""}} -> [w4602]
    shift-right: [w4600] -> _
    shift-left: enum16{"init", "MAIN", "Panel Close"}."init" -> [w4601]
    stop <- w4604 stop-if-true
    # "UNO CODE LOGIC"
    n3529 = case shown="\"MAIN\"" w4601 {
      tunnel: w4606 -> [w4620 w4639 w4695 w4697]
      tunnel: [w4615 w4644 w4695 w4697] -> w4605
      tunnel: [_ _ TRUE _] -> w4604
      tunnel: [w4611 w4642 w4693 w4696] -> w4603
      tunnel: w4602 -> [w4617 w4638 w4693 w4696]
      tunnel: [enum16{"init", "MAIN", "Panel Close"}."MAIN" w4633 _ _] -> w4600
      frame "init" {
        n3530 = local read "Com Port 1"() -> (w4607:refnum<visa-resource-name>)
        n3531 = Bundle By Name(cluster=w4617, "UNO COM Port:"=w4607) -> (w4616:T20)
        n3532 = call "Instrument fgv.vi"("Enum"=T32."INIT", "error in (no error) 2"=w4620, "INPUT"=w4616) -> ("error"=w4618:errorcluster, "output"=w4614:T18)  [unwired: 6 in, 1 out]
        n3533 = case shown="Error" w4618 {
          selector: w4618 -> [w4622 _]
          tunnel: [w4622 w4626] -> w4615
          tunnel: w4614 -> [w4621 w4624]
          tunnel: [w4621 w4623] -> w4612
          frame No Error {
          }
          frame Error {
            n3534 = call "Instrument fgv.vi"("Enum"=T32."ERROR INIT", "INPUT"=w4624) -> ("error"=w4627:errorcluster, "output"=w4623:T18)  [unwired: 7 in, 1 out]
            n3535 = call <vilib>:"Clear Errors.vi"("error in (no error)"=w4627) -> ("error out"=w4626:errorcluster)  [unwired: 5 in, 1 out]
          }
        }
        n3536 = local read "LastCom UNO"() -> (w4609:string)
        n3537 = Unbundle By Name(w4612) -> ("Heave COM Status 2"=→"Instrument Status":bool, "Error Heave"=→"Error  2":errorcluster)  [unwired: 1 out]
        n3538 = Bundle By Name(cluster=w4612, "LastCom"=w4609) -> (w4611:T18)
      }
      frame "MAIN" {
        n3539 = Unbundle By Name(w4638) -> ("UNO COM Port: 2"=w4628:refnum<visa-resource-name>)
        n3540 = local read "Com Port 1"() -> (w4629:refnum<visa-resource-name>)
        n3541 = local write "COM Port UNO :"(w4628) -> ()
        n3542 = Equal?(x=w4628, y=w4629) -> (x = y?=w4645:bool)
        n3543 = Bundle By Name(cluster=w4638, "UNO COM Port:"=w4629) -> (w4637:T20)
        n3544 = case shown="True" w4645 {
          tunnel: [w4649 w4666] -> w4644
          tunnel: w4639 -> [w4650 w4672]
          tunnel: w4637 -> [w4648 w4670]
          tunnel: [w4647 w4665] -> w4642
          frame False {
            n3545 = call <vilib>:"Clear Errors.vi"("error in (no error)"=w4650) -> ("error out"=w4646:errorcluster)  [unwired: 5 in, 1 out]
            n3546 = call "Instrument fgv.vi"("Enum"=T32."ERROR INIT", "error in (no error) 2"=w4646, "INPUT"=w4648) -> ("error"=w4652:errorcluster, "output"=w4647:T18)  [unwired: 6 in, 1 out]
            n3547 = call <vilib>:"Clear Errors.vi"("error in (no error)"=w4652) -> ("error out"=w4649:errorcluster)  [unwired: 5 in, 1 out]
          }
          frame True {
            n3548 = call "Instrument fgv.vi"("Enum"=T32."READ", "error in (no error) 2"=w4672, "INPUT"=w4670) -> ("error"=w4671:errorcluster, "output"=w4664:T18)  [unwired: 6 in, 1 out]
            n3549 = Bundle By Name(cluster=w4664, "String 36"="WRITE UNO") -> (w4663:T18)
            n3550 = case shown="True" "Write" {
              selector: "Write" -> [_ w4687]
              tunnel: w4671 -> [w4685 w4692]
              tunnel: [w4685 w4691] -> w4661
              tunnel: w4663 -> [w4684 w4689]
              tunnel: [w4684 w4688] -> w4660
              frame False {
              }
              frame True {
                n3551 = Not(x=w4687) -> (.not. x?=w4686:bool)
                n3552 = local write "Write"(w4686) -> ()
                n3553 = call "Instrument fgv.vi"("Enum"=T32."MANUAL WRITE", "error in (no error) 2"=w4692, "INPUT"=w4689) -> ("error"=w4691:errorcluster, "output"=w4688:T18)  [unwired: 6 in, 1 out]
              }
            }
            n3554 = Array Size(array="Write UNO") -> (size(s)=w4658:i32)
            n3555 = Greater Than 0?(x=w4658) -> (x > 0?=w4657:bool)
            n3556 = call "Instrument fgv.vi"("Enum"=T32."WRITE", "error in (no error) 2"=w4661, "WriteCC1"="Write UNO", "INPUT"=w4660) -> ("error"=w4668:errorcluster, "WriteCC1 2"=w4659:string[], "output"=w4667:T18)  [unwired: 5 in]
            n3557 = case shown="True" w4657 {
              tunnel: w4659 -> [_ w4674]
              frame False {
              }
              frame True {
                n3558 = local write "Write UNO"(w4674) -> ()
              }
            }
            n3559 = case shown="Error" w4668 {
              selector: w4668 -> [w4675 w4678]
              tunnel: w4667 -> [w4676 w4683]
              tunnel: [w4676 w4682] -> w4665
              tunnel: [w4675 w4680] -> w4666
              frame No Error {
              }
              frame Error {
                n3560 = call <vilib>:"Clear Errors.vi"("error in (no error)"=w4678) -> ("error out"=w4677:errorcluster)  [unwired: 5 in, 1 out]
                n3561 = call "Instrument fgv.vi"("Enum"=T32."ERROR INIT", "error in (no error) 2"=w4677, "INPUT"=w4683) -> ("error"=w4681:errorcluster, "output"=w4682:T18)  [unwired: 6 in, 1 out]
                n3562 = call <vilib>:"Clear Errors.vi"("error in (no error)"=w4681) -> ("error out"=w4680:errorcluster)  [unwired: 5 in, 1 out]
              }
            }
            n3563 = Unbundle By Name(w4665) -> ("LastCom"=→"LastCom UNO":string, "Read Heave and Surge"=→"Read UNO":string)
          }
        }
        n3564 = Unbundle By Name(w4642) -> ("Heave COM Status 2"=w4643:bool, "Heave COM Status"=w4632:bool, "Error Heave"=w4630:errorcluster, "Bytes at Heave Port"=→"Bytes at Humidity Port":dbl)
        n3565 = Not(x=w4632) -> (.not. x?=w4640:bool)
        n3566 = Not(x=w4643) -> (.not. x?=w4631:bool)
        n3567 = local write "Instrument Status"(w4640) -> ()
        n3568 = local write "Error  2"(w4630) -> ()
        n3569 = local write "Port 1a"(w4632) -> ()
        n3570 = local read "Quit"() -> (w4634:bool)
        n3571 = local write "COM Status"(w4631) -> ()
        n3572 = Select(t=enum16{"init", "MAIN", "Panel Close"}."Panel Close", s=w4634, f=enum16{"init", "MAIN", "Panel Close"}."MAIN") -> (s? t:f=w4633:enum16{"init", "MAIN", "Panel Close"})
      }
      frame "Panel Close" {
      }
      frame Default {
      }
    }
  }
